vi "IMAQdx_AbsImage_Flea3_v4.7.vi"() -> ()   [LabVIEW 2013] (continued)
ODTpowBlue(0)\tODTpowXY(DipPowCr)\tvarWaveP1\tProbePow2\tAmp688(depumpPow)\tHalfGaussRamp(t,rMOTpow3,rMOTpow4, BBcompT)\tODTpowX(DipPowX)\tfreq\tHeatingAmp\t0\tSine\tDetuning\tsingleFreqDet\t-20\t8\tDetuning\tsingleFreqStirDet\t0\t0\tBlueBN\tBlueLaserProbeBN\tSSteckBN\tShortSteckDDS\tPixisPos(TOF)\tCycle Wait for Move\t0\t0\t0\t0\t0\t0\t0\t0\t0\t0\t0\t0\t0\t0\t0\t0\t0\t0\t0\t0\t0\t0\t0\t0\r\nBB load\t\tRamp\t0\tloadT\t1\t1\t1\t1\t1\t1\t0\t0\t0\t0\t1\t0\t0\t0\t0\t0\t0\t1\t0\t0\t0\t0\t0\t0\t10u\t1\t1\t0\t0\t0\t0\t1\t1\tplus_zman\tminus_zman\tcompensation\trMOTcurrF\trMOTpow2\tcombAmplitude(combWidthF)\trMOTdelta(-(rMOTbroadDetuningF +combWidthF/2))\tODTpowHLat(DipPowHLat)\t0\t0\t0\t0\t1\t0\t1\t1\t0\tbMOTpow(0.5)\tProbePow\t0\tXshimrMOT\tYshimrMOT\tLineRamp(f,ZshimVar,ZShimVarF)\tODTpowZ(DipPowZ)\t0\t0\t0\t0\t0\t1\t0\t0\t0\t0\t0\t0\t0\t0\t0\t0\t0\t0\trMOTdelta(-(rMOTstirDetF +stirWidthF/2))\tODTpowBlue(0)\tODTpowXY(DipPowCr)\tvarWaveP1\tProbePow2\tAmp688(depumpPow)\trMOTpow4\tODTpowX(DipPowX)\tfreq\tHeatingAmp\t0\tSine\tDetuning\tsingleFreqDet\t-20\t8\tDetuning\tsingleFreqStirDet\t0\t0\tBlueBN\tBlueLaserProbeBN\tSSteckBN\tShortSteckDDS\tPixisPos(TOF)\tCycle Wait for Move\t0\t0\t0\t0\t0\t0\t0\t0\t0\t0\t0\t0\t0\t0\t0\t0\t0\t0\t0\t0\t0\t0\t0\t0\r\nSF\t\tRamp\t1\tSFcoolT\t0\t0\t1\t1\t1\t1\t0\t0\t0\t1\t1\t0\t0\t0\t0\t0\t0\t1\t0\t0\t0\t0\t0\t0\t10u\t1\t1\t0\t0\t0\t0\t1\t1\tplus_zman\tminus_zman\tcompensation\trMOTcurrF\trMOTpow2\tcombAmplitude(combWidthF)\trMOTdelta(-(rMOTbroadDetuningF +combWidthF/2))\tODTpowHLat(DipPowHLat)\t0\t0\t0\t0\t1\t0\t1\t1\t0\tbMOTpow(0.5)\tProbePow\t0\tXshimrMOT\tYshimrMOT\tZshimVar\tODTpowZ(DipPowZ)\t0\t0\t0\t0\t0\t1\t0\t0\t0\t0\t0\t0\t0\t0\t0\t0\t0\t0\trMOTdelta(-(rMOTstirDetF +stirWidthF/2))\tODTpowBlue(0)\tODTpowXY(DipPowCr)\tvarWaveP1\tProbePow2\tAmp688(depumpPow)\trMOTpow4\tODTpowX(DipPowX)\tfreq\tHeatingAmp\t0\tSine\tRamp\tsingleFreqDet\tsingleFreqDet + SFramp\tSFcoolT*1000\tRamp\tsingleFreqStirDet\tsingleFreqStirDet + SFramp\tSFcoolT*1000\tBlueBN\tBlueLaserProbeBN\tSSteckBN\tShortSteckDDS\tPixisPos(TOF)\tCycle Wait for Move\t0\t0\t0\t0\t0\t0\t0\t0\t0\t0\t0\t0\t0\t0\t0\t0\t0\t0\t0\t0\t0\t0\t0\t0\r\nload1\t\tRamp\t1\tloadT\t0\t0\t1\t1\t1\t1\t1\t0\t1\t1\t1\t0\t0\t1\t0\t0\t0\t1\t0\t0\t0\t0\t0\t0\t10u\t1\t1\t0\t0\t0\t0\t1\t1\tplus_zman\tminus_zman\tcompensation\trMOTcurrF\tLineRamp(f,rMOTpow2,rMOTpow5)\tcombAmplitude(combWidthF)\trMOTdelta(-(rMOTbroadDetuningF +combWidthF/2))\tODTpowHLat(DipPowHLat)\t0\t0\t0\t0\t1\t0\t1\t1\t0\tbMOTpow(0.5)\tProbePow\t0\tXshimrMOT\tYshimrMOT\tLineRamp(f,ZshimVar,ZShimVarF)\tODTpowZ(DipPowZ)\t0\t0\t0\t0\t0\t1\t0\t1\t0\t0\t0\t0\t0\t0\t0\t0\t0\t0\trMOTdelta(-(rMOTstirDetF +stirWidthF/2))\tODTpowBlue(0)\tODTpowXY(DipPowCr)\tvarWaveP1\tProbePow2\tAmp688(depumpPow)\tLineRamp(f,rMOTpow4,rMOTpow6)\tODTpowX(DipPowX)\tfreq\tHeatingAmp\t0\tSine\tRamp\tsingleFreqDet +SFramp\tsingleFreqDet + SFramp + SFramp2\tloadT*1000\tRamp\tsingleFreqStirDet + SFramp\tsingleFreqStirDet + SFramp + SFramp2\tloadT*1000\tBlueBN\tBlueLaserProbeBN\tSSteckBN\tShortSteckDDS\tPixisPos(TOF)\tCycle Wait for Move\t0\t0\t0\t0\t0\t0\t0\t0\t0\t0\t0\t0\t0\t0\t0\t0\t0\t0\t0\t0\t0\t0\t0\t0\r\nload2\t\tRamp\t0\t.05\t1\t1\t1\t1\t1\t1\t0\t0\t1\t1\t1\t0\t0\t1\t0\t0\t0\t1\t0\t0\t0\t0\t0\t0\t0\t1\t1\t0\t0\t0\t0\t1\t1\tplus_zman\tminus_zman\tcompensation\trMOTcurrF\trMOTpow5\tcombAmplitude(combWidthF)\trMOTdelta(-(rMOTbroadDetuningF +combWidthF/2))\tODTpowHLat(DipPowHLat)\t0\t0\t0\t0\t1\t0\t1\t1\t0\tbMOTpow(0.5)\tProbePow\t0\tXshimrMOT\tYshimrMOT\tZshimVar\tODTpowZ(DipPowZ)\t0\t0\t0\t0\t0\t1\t0\t0\t0\t0\t0\t0\t0\t0\t0\t0\t0\t0\trMOTdelta(-(rMOTstirDetF +stirWidthF/2))\tODTpowBlue(0)\tODTpowXY(DipPowCr)\tvarWaveP1\tProbePow2\tAmp688(depumpPow)\trMOTpow6\tODTpowX(DipPowX)\tfreq\tHeatingAmp\t0\tSine\tDetuning\tsingleFreqDet +SFramp\tsingleFreqDet + SFramp + SFramp2\tloadT*1000\tDetuning\tsingleFreqStirDet + SFramp\tsingleFreqStirDet + SFramp + SFramp2\tloadT*1000\tBlueBN\tBlueLaserProbeBN\tSSteckBN\tShortSteckDDS\tPixisPos(TOF)\tCycle Wait for Move\t0\t0\t0\t0\t0\t0\t0\t0\t0\t0\t0\t0\t0\t0\t0\t0\t0\t0\t0\t0\t0\t0\t0\t0\r\ndrop Red MOT\t\tRamp\t0\t.045\t1\t1\t1\t1\t1\t1\t0\t0\t1\t1\t0\t0\t0\t1\t0\t0\t0\t1\t0\t0\t0\t0\t0\t0\t0\t1\t1\t0\t0\t0\t1\t1\t0\tplus_zman\tminus_zman\tcompensation\trMOTcurrF\trMOTpow5\tcombAmplitude(combWidthF)\trMOTdelta(-(rMOTbroadDetuningF +combWidthF/2))\tODTpowHLat(0.3)\t0\t0\t0\t0\t1\t0\t1\t1\t0\tbMOTpow(0.5)\tProbePow\t0\tXshimrMOT\tYshimrMOT\tZShimVarF\tODTpowZ(DipPowZ)\t0\t0\t0\t0\t0\t1\t0\t1\t0\t0\t0\t0\t0\t0\t0\t0\t0\t0\trMOTdelta(-(rMOTstirDetF +stirWidthF/2))\tODTpowBlue(0)\tODTpowXY(DipPowCr)\tvarWaveP1\tProbePow2\tAmp688(depumpPow)\trMOTpow6\tODTpowX(DipPowX)\tfreq\tHeatingAmp\t0\tSine\tDetuning\tDoppCoolDet\tsingleFreqDet + SFramp + SFramp2\tloadT*1000\tDetuning\tDoppCoolStirDet\tsingleFreqStirDet + SFramp + SFramp2\tloadT*1000\tBlueBN\tBlueLaserProbeBN\tSSteckBN\tShortSteckDDS\tPixisPos(TOF)\tCycle Wait for Move\t0\t0\t0\t0\t0\t0\t0\t0\t0\t0\t0\t0\t0\t0\t0\t0\t0\t0\t0\t0\t0\t0\t0\t0\r\nramp Trap\t\tRamp\t1\trampT\t0\t0\t1\t1\t1\t1\t0\t0\t1\t1\t0\t0\t0\t1\t0\t0\t0\t1\t0\t0\t0\t0\t0\t0\t10u\t1\t1\t0\t0\t0\t1\t1\t0\tplus_zman\tminus_zman\tcompensation\trMOTcurrF\trMOTpow3\tcombAmplitude(combWidthF)\trMOTdelta(-(rMOTbroadDetuningF +combWidthF/2))\tODTpowHLat(DipPowHLat)\t0\t0\t0\t0\t1\t0\t1\t1\t0\tbMOTpow(0.5)\tProbePow\t0\tXshimDC\tYshimDC\tZshimDC\tSinRamp(t,(ODTpowZ(DipPowZ)+ODTpowZ(DipPowZ2))/2,(ODTpowZ(DipPowZ2)-ODTpowZ(DipPowZ))/2,1/(2*rampT),3*pi/2)\t0\t0\t0\t0\t0\t1\t0\t0\t0\t0\t0\t0\t0\t0\t0\t0\t0\t0\trMOTdelta(-(rMOTstirDetI +stirWidthF/2))\tODTpowBlue(0)\tSinRamp(t,(ODTpowXY(DipPowCr)+ODTpowXY(DipPowCr2))/2,(ODTpowXY(DipPowCr2)-ODTpowXY(DipPowCr))/2,1/(2*rampT),3*pi/2)\tvarWaveP1\tProbePow2\tAmp688(depumpPow)\trMOTpow6\tSinRamp(t,(ODTpowX(DipPowX)+ODTpowX(DipPowX2))/2,(ODTpowX(DipPowX2)-ODTpowX(DipPowX))/2,1/(2*rampT),3*pi/2)\tfreq\tHeatingAmp\t0\tSine\tDetuning\tsingleFreqDetF\tsingleFreqDet + SFramp + SFramp2\tloadT*1000\tDetuning\tsingleFreqStirDetF\tsingleFreqStirDet + SFramp + SFramp2\tloadT*1000\tBlueBN\tBlueLaserProbeBN\tSSteckBN\tShortSteckDDS\tPixisPos(TOF)\tCycle Wait for Move\t0\t0\t0\t0\t0\t0\t0\t0\t0\t0\t0\t0\t0\t0\t0\t0\t0\t0\t0\t0\t0\t0\t0\t0\r\nhold\t\tRamp\t0\t.01\t1\t1\t1\t1\t1\t1\t0\t0\t1\t1\t0\t0\t0\t1\t0\t0\t0\t1\t0\t0\t0\t0\t0\t0\t0\t1\t1\t0\t0\t0\t1\t1\t0\tplus_zman\tminus_zman\tcompensation\trMOTcurrF\trMOTpow4\tcombAmplitude(combWidthF)\trMOTdelta(-(rMOTbroadDetuningF +combWidthF/2))\tODTpowHLat(DipPowHLat)\t0\t0\t0\t0\t1\t0\t1\t1\t0\tbMOTpow(0.5)\tProbePow\t0\tXshimDC\tYshimDC\tZshimDC\tODTpowZ(DipPowZ2)\t0\t0\t0\t0\t0\t1\t0\t0\t0\t0\t0\t0\t0\t0\t0\t0\t0\t0\trMOTdelta(-(rMOTstirDetI +stirWidthF/2))\tODTpowBlue(0)\tODTpowXY(DipPowCr2)\tvarWaveP1\tProbePow2\tAmp688(depumpPow)\trMOTpow6\tODTpowX(DipPowX2)\tfreq\tHeatingAmp\t0\tSine\tDetuning\tDoppCoolDetF\tsingleFreqDet + SFramp + SFramp2\tloadT*1000\tDetuning\tDoppCoolStirDet\tsingleFreqStirDet + SFramp + SFramp2\tloadT*1000\tBlueBN\tBlueLaserProbeBN\tSSteckBN\tShortSteckDDS\tPixisPos(TOF)\tCycle Wait for Move\t0\t0\t0\t0\t0\t0\t0\t0\t0\t0\t0\t0\t0\t0\t0\t0\t0\t0\t0\t0\t0\t0\t0\t0\r\nramp Trap\t\tRamp\t0\trampT\t1\t1\t1\t1\t1\t1\t0\t0\t1\t1\t0\t0\t0\t1\t0\t0\t0\t1\t0\t0\t0\t0\t0\t0\t10u\t1\t1\t0\t0\t0\t1\t1\t0\tplus_zman\tminus_zman\tcompensation\trMOTcurrF\trMOTpow3\tcombAmplitude(combWidthF)\trMOTdelta(-(rMOTbroadDetuningF +combWidthF/2))\tODTpowHLat(DipPowHLat)\t0\t0\t0\t0\t1\t0\t1\t1\t0\tbMOTpow(0.5)\tProbePow\t0\tXshimDC\tYshimDC\tZshimDC\tSinRamp(t,(ODTpowZ(DipPowZ)+ODTpowZ(DipPowZ2))/2,(ODTpowZ(DipPowZ2)-ODTpowZ(DipPowZ))/2,1/(2*rampT),pi/2)\t0\t0\t0\t0\t0\t1\t0\t0\t0\t0\t0\t0\t0\t0\t0\t0\t0\t0\trMOTdelta(-(rMOTstirDetI +stirWidthF/2))\tODTpowBlue(0)\tSinRamp(t,(ODTpowXY(DipPowCr)+ODTpowXY(DipPowCr2))/2,(ODTpowXY(DipPowCr2)-ODTpowXY(DipPowCr))/2,1/(2*rampT),pi/2)\tvarWaveP1\tProbePow2\tAmp688(depumpPow)\trMOTpow6\tSinRamp(t,(ODTpowX(DipPowX)+ODTpowX(DipPowX2))/2,(ODTpowX(DipPowX2)-ODTpowX(DipPowX))/2,1/(2*rampT),pi/2)\tfreq\tHeatingAmp\t0\tSine\tDetuning\tsingleFreqDetF\tsingleFreqDet + SFramp + SFramp2\tloadT*1000\tDetuning\tsingleFreqStirDetF\tsingleFreqStirDet + SFramp + SFramp2\tloadT*1000\tBlueBN\tBlueLaserProbeBN\tSSteckBN\tShortSteckDDS\tPixisPos(TOF)\tCycle Wait for Move\t0\t0\t0\t0\t0\t0\t0\t0\t0\t0\t0\t0\t0\t0\t0\t0\t0\t0\t0\t0\t0\t0\t0\t0\r\nhold\t\tRamp\t0\t.5\t1\t1\t1\t1\t1\t1\t0\t0\t1\t1\t0\t0\t0\t1\t0\t0\t0\t1\t0\t0\t0\t0\t0\t0\t0\t1\t1\t0\t0\t0\t1\t1\t0\tplus_zman\tminus_zman\tcompensation\trMOTcurrF\trMOTpow4\tcombAmplitude(combWidthF)\trMOTdelta(-(rMOTbroadDetuningF +combWidthF/2))\tODTpowHLat(DipPowHLat)\t0\t0\t0\t0\t1\t0\t1\t1\t0\tbMOTpow(0.5)\tProbePow\t0\tXshimDC\tYshimDC\tZshimDC\tODTpowZ(DipPowZ)\t0\t0\t0\t0\t0\t1\t0\t0\t0\t0\t0\t0\t0\t0\t0\t0\t0\t0\trMOTdelta(-(rMOTstirDetI +stirWidthF/2))\tODTpowBlue(0)\tODTpowXY(DipPowCr)\tvarWaveP1\tProbePow2\tAmp688(depumpPow)\trMOTpow6\tODTpowX(DipPowX)\tfreq\tHeatingAmp\t0\tSine\tDetuning\tDoppCoolDetF\tsingleFreqDet + SFramp + SFramp2\tloadT*1000\tDetuning\tDoppCoolStirDet\tsingleFreqStirDet + SFramp + SFramp2\tloadT*1000\tBlueBN\tBlueLaserProbeBN\tSSteckBN\tShortSteckDDS\tPixisPos(TOF)\tCycle Wait for Move\t0\t0\t0\t0\t0\t0\t0\t0\t0\t0\t0\t0\t0\t0\t0\t0\t0\t0\t0\t0\t0\t0\t0\t0\r\nDoppler Cool1\t\tRamp\t0\tdopCoolT\t1\t1\t1\t1\t1\t1\t0\t0\t1\t1\t1\t0\t0\t1\t0\t0\t0\t1\t0\t0\t0\t0\t0\t0\t10u\t1\t1\t0\t0\t0\t1\t1\t1\tplus_zman\tminus_zman\tcompensation\trMOTcurrF\tDoppCoolPow\tcombAmplitude(combWidthF)\trMOTdelta(-(rMOTbroadDetuningF +combWidthF/2))\tODTpowHLat(DipPowHLat)\t0\t0\t0\t0\t1\t0\t1\t1\t0\tbMOTpow(0.5)\tProbePow\t0\tXshimDC\tYshimDC\tZshimDC\tODTpowZ(DipPowZ)\t0\t0\t0\t0\t0\t1\t0\t0\t0\t0\t0\t0\t0\t0\t0\t0\t0\t0\trMOTdelta(-(rMOTstirDetI +stirWidthF/2))\tODTpowBlue(0)\tODTpowXY(DipPowCr)\tvarWaveP1\tProbePow2\tAmp688(depumpPow)\tDoppStirPow\tODTpowX(DipPowX2)\tfreq\tHeatingAmp\t0\tSine\tDetuning\tDoppCoolDet\tsingleFreqDet + SFramp + SFramp2\tloadT*1000\tDetuning\tDoppCoolStirDet\tsingleFreqStirDet + SFramp + SFramp2\tloadT*1000\tBlueBN\tBlueLaserProbeBN\tSSteckBN\tShortSteckDDS\tPixisPos(TOF)\tCycle Wait for Move\t0\t0\t0\t0\t0\t0\t0\t0\t0\t0\t0\t0\t0\t0\t0\t0\t0\t0\t0\t0\t0\t0\t0\t0\r\nDoppler Cool2\t\tRamp\t0\tdopCoolT\t1\t1\t1\t1\t1\t1\t0\t0\t1\t1\t1\t0\t0\t1\t0\t0\t0\t1\t0\t0\t0\t0\t0\t0\t10u\t1\t1\t0\t0\t0\t1\t1\t1\tplus_zman\tminus_zman\tcompensation\trMOTcurrF\trMOTpow5\tcombAmplitude(combWidthF)\trMOTdelta(-(rMOTbroadDetuningF +combWidthF/2))\tODTpowHLat(DipPowHLat)\t0\t0\t0\t0\t1\t0\t1\t1\t0\tbMOTpow(0.5)\tProbePow\t0\tXshimDC\tYshimDC\tZshimDC\tODTpowZ(DipPowZ)\t0\t0\t0\t0\t0\t1\t0\t0\t0\t0\t0\t0\t0\t0\t0\t0\t0\t0\trMOTdelta(-(rMOTstirDetI +stirWidthF/2))\tODTpowBlue(0)\tODTpowXY(DipPowCr)\tvarWaveP1\tProbePow2\tAmp688(depumpPow)\trMOTpow6\tODTpowX(DipPowX2)\tfreq\tHeatingAmp\t0\tSine\tRamp\tDoppCoolDet\tDoppCoolDet-DoppCoolSweep\tdopCoolT*1000\tDetuning\tDoppCoolStirDet\tsingleFreqStirDet + SFramp + SFramp2\tloadT*1000\tBlueBN\tBlueLaserProbeBN\tSSteckBN\tShortSteckDDS\tPixisPos(TOF)\tCycle Wait for Move\t0\t0\t0\t0\t0\t0\t0\t0\t0\t0\t0\t0\t0\t0\t0\t0\t0\t0\t0\t0\t0\t0\t0\t0\r\nDoppler Cool3\t\tRamp\t0\tdopCoolT\t1\t1\t1\t1\t1\t1\t0\t0\t1\t1\t1\t0\t0\t1\t0\t0\t0\t1\t0\t0\t0\t0\t0\t0\t10u\t1\t1\t0\t0\t0\t1\t1\t1\tplus_zman\tminus_zman\tcompensation\trMOTcurrF\tLineRamp(f,rMOTpow4,rMOTpow5)\tcombAmplitude(combWidthF)\trMOTdelta(-(rMOTbroadDetuningF +combWidthF/2))\tODTpowHLat(DipPowHLat)\t0\t0\t0\t0\t1\t0\t1\t1\t0\tbMOTpow(0.5)\tProbePow\t0\tXshimDC\tYshimDC\tZshimDC\tODTpowZ(DipPowZ)\t0\t0\t0\t0\t0\t1\t0\t0\t0\t0\t0\t0\t0\t0\t0\t0\t0\t0\trMOTdelta(-(rMOTstirDetI +stirWidthF/2))\tODTpowBlue(0)\tODTpowXY(DipPowCr)\tvarWaveP1\tProbePow2\tAmp688(depumpPow)\tLineRamp(f,rMOTpow4,rMOTpow5)\tODTpowX(DipPowX2)\tfreq\tHeatingAmp\t0\tSine\tDetuning\tDoppCoolDet-DoppCoolSweep\tDoppCoolDet-DoppCoolSweep\tdopCoolT*1000\tDetuning\tDoppCoolStirDet\tsingleFreqStirDet + SFramp + SFramp2\tloadT*1000\tBlueBN\tBlueLaserProbeBN\tSSteckBN\tShortSteckDDS\tPixisPos(TOF)\tCycle Wait for Move\t0\t0\t0\t0\t0\t0\t0\t0\t0\t0\t0\t0\t0\t0\t0\t0\t0\t0\t0\t0\t0\t0\t0\t0\r\nhold\t\tRamp\t0\t2\t1\t1\t0\t0\t0\t0\t0\t0\t1\t1\t0\t0\t0\t1\t0\t0\t0\t1\t0\t0\t0\t0\t0\t0\t0\t1\t1\t0\t0\t0\t1\t1\t0\tplus_zman\tminus_zman\tcompensation\trMOTcurrF\trMOTpow4\tcombAmplitude(combWidthF)\trMOTdelta(-(rMOTbroadDetuningF +combWidthF/2))\tODTpowHLat(DipPowHLat)\t0\t0\t0\t0\t1\t0\t1\t1\t0\tbMOTpow(0.5)\tProbePow\t0\tXshimrMOT\tYshimrMOT\tZshimVar\tODTpowZ(DipPowZ)\t0\t0\t0\t0\t0\t1\t0\t0\t0\t0\t0\t0\t0\t0\t0\t0\t0\t0\trMOTdelta(-(rMOTstirDetI +stirWidthF/2))\tODTpowBlue(0)\tODTpowXY(DipPowCr2)\tvarWaveP1\tProbePow2\tAmp688(depumpPow)\trMOTpow4\tLineRamp(f, ODTpowX(DipPowX), ODTpowX(DipPowX2))\tfreq\tHeatingAmp\t0\tSine\tDetuning\tDoppCoolDet-DoppCoolSweep\tDoppCoolDet-DoppCoolSweep\tdopCoolT*1000\tDetuning\tDoppCoolStirDet\tsingleFreqStirDet + SFramp + SFramp2\tloadT*1000\tBlueBN\tBlueLaserProbeBN\tSSteckBN\tShortSteckDDS\tPixisPos(TOF)\tCycle Wait for Move\t0\t0\t0\t0\t0\t0\t0\t0\t0\t0\t0\t0\t0\t0\t0\t0\t0\t0\t0\t0\t0\t0\t0\t0\r\nhold\t\tRamp\t0\tholdT\t1\t1\t0\t0\t0\t0\t0\t0\t1\t1\t0\t0\t0\t1\t0\t0\t0\t1\t0\t0\t0\t0\t0\t0\t0\t1\t1\t0\t0\t0\t1\t1\t0\tplus_zman\tminus_zman\tcompensation\trMOTcurrF\trMOTpow4\tcombAmplitude(combWidthF)\trMOTdelta(-(rMOTbroadDetuningF +combWidthF/2))\tODTpowHLat(DipPowHLat2)\t0\t0\t0\t0\t1\t0\t1\t1\t0\tbMOTpow(0.5)\tProbePow\t0\tXshimrMOT\tYshimrMOT\tZshimVar\tODTpowZ(DipPowZ)\t0\t0\t0\t0\t0\t1\t0\t0\t0\t0\t0\t0\t0\t0\t0\t0\t0\t0\trMOTdelta(-(rMOTstirDetI +stirWidthF/2))\tODTpowBlue(0)\tODTpowXY(DipPowCr)\tvarWaveP1\tProbePow2\tAmp688(depumpPow)\trMOTpow4\tODTpowX(DipPowX)\tfreq\tHeatingAmp\t0\tSine\tDetuning\tDoppCoolDet-DoppCoolSweep\tDoppCoolDet-DoppCoolSweep\tdopCoolT*1000\tDetuning\tDoppCoolStirDet\tsingleFreqStirDet + SFramp + SFramp2\tloadT*1000\tBlueBN\tBlueLaserProbeBN\tSSteckBN\tShortSteckDDS\tPixisPos(TOF)\tCycle Wait for Move\t0\t0\t0\t0\t0\t0\t0\t0\t0\t0\t0\t0\t0\t0\t0\t0\t0\t0\t0\t0\t0\t0\t0\t0\r\ndrop HTrap\t\tRamp\t0\t.03\t1\t1\t1\t1\t1\t1\t0\t0\t1\t1\t0\t0\t0\t1\t0\t0\t0\t1\t0\t0\t0\t0\t0\t0\t0\t1\t1\t0\t0\t0\t1\t1\t0\tplus_zman\tminus_zman\tcompensation\trMOTcurrF\trMOTpow3\tcombAmplitude(combWidthF)\trMOTdelta(-(rMOTbroadDetuningF +combWidthF/2))\tODTpowHLat(DipPowHLat)\t0\t0\t0\t0\t1\t0\t1\t1\t0\tbMOTpow(0.5)\tProbePow\t0\tXshimrMOT\tYshimrMOT\tZshimVar\tODTpowZ(DipPowZ)\t0\t0\t0\t0\t0\t1\t0\t0\t0\t0\t0\t0\t0\t0\t0\t0\t0\t0\trMOTdelta(-(rMOTstirDetI +stirWidthF/2))\tODTpowBlue(0)\tODTpowXY(DipPowCr)\tvarWaveP1\tProbePow2\tAmp688(depumpPow)\trMOTpow3\tODTpowX(DipPowX)\tfreq\tHeatingAmp\t0\tSine\tDetuning\tsingleFreqDet +20\tDoppCoolDet-DoppCoolSweep\tdopCoolT*1000\tDetuning\tsingleFreqStirDet + 20\tsingleFreqStirDet + SFramp + SFramp2\tloadT*1000\tBlueBN\tBlueLaserProbeBN\tSSteckBN\tShortSteckDDS\tPixisPos(TOF)\tCycle Wait for Move\t0\t0\t0\t0\t0\t0\t0\t0\t0\t0\t0\t0\t0\t0\t0\t0\t0\t0\t0\t0\t0\t0\t0\t0\r\nmodulate\t\tRamp\t0\t3m\t1\t1\t1\t1\t1\t1\t0\t0\t1\t1\t0\t0\t0\t1\t0\t0\t0\t1\t0\t0\t0\t0\t0\t0\t0\t1\t1\t0\t0\t0\t1\t1\t0\tplus_zman\tminus_zman\tcompensation\trMOTcurrF\trMOTpow3\tcombAmplitude(combWidthF)\trMOTdelta(-(rMOTbroadDetuningF +combWidthF/2))\tODTpowHLat(DipPowHLat)\t0\t0\t0\t0\t1\t0\t1\t1\t0\tbMOTpow(0.5)\tProbePow\t0\tXshimrMOT\tYshimrMOT\tZshimVar\tODTpowZ(DipPowZ)\t0\t0\t0\t0\t0\t1\t0\t0\t0\t0\t0\t0\t0\t0\t0\t0\t0\t0\trMOTdelta(-(rMOTstirDetI +stirWidthF/2))\tODTpowBlue(0)\tODTpowXY(DipPowCr)\tvarWaveP1\tProbePow2\tAmp688(depumpPow)\trMOTpow3\tODTpowX(DipPowX)\tfreq\tHeatingAmp\t0\tSine\tDetuning\tsingleFreqDet +20\tDoppCoolDet-DoppCoolSweep\tdopCoolT*1000\tDetuning\tsingleFreqStirDet + 20\tsingleFreqStirDet + SFramp + SFramp2\tloadT*1000\tBlueBN\tBlueLaserProbeBN\tSSteckBN\tShortSteckDDS\tPixisPos(TOF)\tCycle Wait for Move\t0\t0\t0\t0\t0\t0\t0\t0\t0\t0\t0\t0\t0\t0\t0\t0\t0\t0\t0\t0\t0\t0\t0\t0\r\nEvaporation\t\tRamp\tevapOn\ttEvap1\t0\t0\t1\t1\t1\t1\t0\t0\t1\t1\t0\t0\t0\t1\t0\t0\t0\t1\t0\t0\t0\t0\t0\t0\t1m\t1\t1\t0\t0\t0\t1\t1\t0\tplus_zman\tminus_zman\tcompensation\trMOTcurrF\trMOTpow3\tcombAmplitude(combWidthF)\trMOTdelta(-(rMOTbroadDetuningF +combWidthF/2))\tODTpowHLat(DipPowHLat)\t0\t0\t0\t0\t1\t0\t1\t1\t0\tbMOTpow(0.5)\tProbePow\t0\tXshimrMOT\tYshimrMOT\tZshimVar\tLineRamp(f,ODTpowZ(DipPowZ2),ODTpowZ(DipPowZ3))\t0\t0\t0\t0\t0\t1\t0\t1\t0\t0\t0\t0\t0\t0\t0\t0\t0\t0\trMOTdelta(-(rMOTstirDetI +stirWidthF/2))\tODTpowBlue(0)\tExpRamp2(t,0,ODTpowXY(DipPowCr2),ODTpowXY(DipPowCr3),tau)\tvarWaveP1\tProbePow2\tAmp688(depumpPow)\trMOTpow3\tExpRamp2(t,0,ODTpowX(DipPowX2),ODTpowX(DipPowX3),tau)\tfreq\tHeatingAmp\t0\tSine\tDetuning\tsingleFreqDet +20\tDoppCoolDet-DoppCoolSweep\tdopCoolT*1000\tDetuning\tsingleFreqStirDet + 20\tsingleFreqStirDet + SFramp + SFramp2\tloadT*1000\tBlueBN\tBlueLaserProbeBN\tSSteckBN\tShortSteckDDS\tPixisPos(TOF)\tCycle Wait for Move\t0\t0\t0\t0\t0\t0\t0\t0\t0\t0\t0\t0\t0\t0\t0\t0\t0\t0\t0\t0\t0\t0\t0\t0\r\npost evap hold\t\tRamp\t1\tholdT\t1\t1\t1\t1\t1\t1\t0\t0\t1\t1\t0\t0\t0\t1\t0\t0\t0\t1\t0\t0\t0\t0\t0\t0\t0\t1\t1\t0\t0\t0\t1\t1\t0\tplus_zman\tminus_zman\tcompensation\trMOTcurrF\trMOTpow3\tcombAmplitude(combWidthF)\trMOTdelta(-(rMOTbroadDetuningF +combWidthF/2))\tODTpowHLat(DipPowHLat2)\t0\t0\t0\t0\t1\t0\t1\t1\t0\tbMOTpow(0.5)\tProbePow\t0\tXshimrMOT\tYshimrMOT\tZshimVar\tODTpowZ(DipPowZ3)\t1\t0\t0\t0\t0\t1\t0\t1\t0\t0\t0\t0\t0\t0\t0\t0\t0\t0\trMOTdelta(-(rMOTstirDetI +stirWidthF/2))\tODTpowBlue(0)\tExpFinal(tEvap1,ODTpowXY(DipPowCr2),ODTpowXY(DipPowCr3),tau)\tvarWaveP1\tProbePow2\tAmp688(depumpPow)\trMOTpow3\tExpFinal(tEvap1,ODTpowX(DipPowX2),ODTpowX(DipPowX3),tau)\tfreq\tHeatingAmp\t0\tSine\tDetuning\tsingleFreqDet +20\tDoppCoolDet-DoppCoolSweep\tdopCoolT*1000\tDetuning\tsingleFreqStirDet + 20\tsingleFreqStirDet + SFramp + SFramp2\tloadT*1000\tBlueBN\tBlueLaserProbeBN\tSSteckBN\tShortSteckDDS\tPixisPos(TOF)\tCycle Wait for Move\t0\t0\t0\t0\t0\t0\t0\t0\t0\t0\t0\t0\t0\t0\t0\t0\t0\t0\t0\t0\t0\t0\t0\t0\r\nbox ramp up\t\tRamp\t0\tboxLoadT\t0\t0\t1\t1\t1\t1\t0\t0\t1\t1\t0\t0\t0\t1\t0\t0\t0\t1\t0\t0\t0\t0\t0\t0\t1m\t1\t1\t0\t0\t0\t1\t1\t0\tplus_zman\tminus_zman\tcompensation\trMOTcurrF\trMOTpow3\tcombAmplitude(combWidthF)\trMOTdelta(-(rMOTbroadDetuningF +combWidthF/2))\tODTpowHLat(DipPowHLat)\t0\t0\t0\t0\t1\t0\t1\t1\tpulseTTL(f,94)\tbMOTpow(0.5)\tProbePow\t0\tXshimrMOT\tYshimrMOT\tZshimVar\tODTpowZ(DipPowZ3)\t0\t0\tboxOn\t0\t0\t1\t0\t0\t0\t0\t0\t0\t0\t0\t0\t0\t0\t0\trMOTdelta(-(rMOTstirDetI +stirWidthF/2))\tSinRamp(t,(ODTpowBlue(BlueDipPow)+ODTpowBlue(0))/2,(ODTpowBlue(BlueDipPow)-ODTpowBlue(0))/2,1/(2*boxLoadT),3*pi/2)\tExpFinal(tEvap1,ODTpowXY(DipPowCr2),ODTpowXY(DipPowCr3),tau)\tvarWaveP1\tProbePow2\tAmp688(depumpPow)\trMOTpow3\tExpFinal(tEvap1,ODTpowX(DipPowX2),ODTpowX(DipPowX3),tau)\tfreq\tHeatingAmp\t0\tSine\tDetuning\tsingleFreqDet +20\tDoppCoolDet-DoppCoolSweep\tdopCoolT*1000\tDetuning\tsingleFreqStirDet + 20\tsingleFreqStirDet + SFramp + SFramp2\tloadT*1000\tBlueBN\tBlueLaserProbeBN\tSSteckBN\tShortSteckDDS\tPixisPos(TOF)\tCycle Wait for Move\t0\t0\t0\t0\t0\t0\t0\t0\t0\t0\t0\t0\t0\t0\t0\t0\t0\t0\t0\t0\t0\t0\t0\t0\r\nbox lat ramp up\t\tRamp\t0\tboxLoadT\t1\t1\t1\t1\t1\t1\t0\t0\t1\t1\t0\t0\t0\t1\t0\t0\t0\t1\t0\t0\t0\t0\t0\t0\t1m\t1\t1\t0\t0\t0\t1\t1\t0\tplus_zman\tminus_zman\tcompensation\trMOTcurrF\trMOTpow3\tcombAmplitude(combWidthF)\trMOTdelta(-(rMOTbroadDetuningF +combWidthF/2))\tSinRamp(t,(ODTpowHLat(DipPowHLat)+ODTpowHLat(DipPowHLat2))/2,(ODTpowHLat(DipPowHLat)-ODTpowHLat(DipPowHLat2))/2,1/(2*rampLatT), pi/2)\t0\t0\t0\t0\t1\t0\t1\t1\tpulseTTL(f,94)\tbMOTpow(0.5)\tProbePow\t0\tXshimrMOT\tYshimrMOT\tZshimVar\tSinRamp(t,(ODTpowZ(DipPowZ3)+ODTpowZ(DipPowZLat))/2, (ODTpowZ(DipPowZ3)-ODTpowZ(DipPowZLat))/2, 1/(2*rampLatT), pi/2)\t0\t0\tboxOn\t0\t1\t1\t0\t0\t0\t0\t0\t0\t0\t0\t0\t0\t0\t0\trMOTdelta(-(rMOTstirDetI +stirWidthF/2))\tSinRamp(t,(ODTpowBlue(BlueDipPow)+ODTpowBlue(0))/2,(ODTpowBlue(BlueDipPow)-ODTpowBlue(0))/2,1/(2*boxLoadT),3*pi/2)\tExpFinal(tEvap1,ODTpowXY(DipPowCr2),ODTpowXY(DipPowCr3),tau)\tLineRamp(f,varWaveP1,varWaveP2)\tProbePow2\tAmp688(depumpPow)\t